vi "FlexMag - 24-03-2023.vi"() -> ()   [LabVIEW 2018] (continued)
                    n11930 = local read "ABORT"() -> (w17188:bool)
                    n11931 = case shown="False" w17188 {
                      frame False {
                        n11932 = while {
                          i -> [w17193]
                          stop <- w17194 stop-if-true
                          n11933 = Greater Or Equal?(x=w17193, y=100) -> (x >= y?=w17191:bool)
                          n11934 = case shown="True" w17191 {
                            frame False {
                            }
                            frame True {
                              n11935 = local write "Warning Message"("Transfer process canceled!\nCH3 Trns Bp Right coulnt't be closed" ("Warning Message")) -> ()
                              n11936 = local write "trns error"(TRUE ("TRNS error")) -> ()
                            }
                          }
                          n11937 = local read "CH3_Trns_BP_Right_DI"() -> (w17189:bool)
                          n11938 = case shown="True" w17189 {
                            tunnel: [TRUE ("CH1_Trns_BP_Left_DO") FALSE ("CH1_Trns_BP_Left_DO")] -> w17190
                            frame False {
                            }
                            frame True {
                              n11939 = local write "CH3_Trns_BP_Right_DO"(FALSE ("TRNS error")) -> ()
                              n11940 = Wait Until Next ms Multiple(millisecond multiple=u32 200) -> ()  [unwired: 1 out]
                            }
                          }
                          n11941 = local read "ch3-2 transfer"() -> (w17197:bool)
                          n11942 = local read "ABORT"() -> (w17196:bool)
                          n11943 = Not(x=w17197) -> (.not. x?=w17195:bool)
                          n11944 = Compound Arithmetic op=OR(w17190, w17196, w17195) -> (w17194:bool)
                        }
                      }
                      frame True {
                      }
                    }
                  }
                }
              }
              frame #43 {
                n11945 = local read "ch3-2 transfer"() -> (w17204:bool)
                n11946 = case shown="True" w17204 {
                  frame False {
                  }
                  frame True {
                    n11947 = local read "ABORT"() -> (w17205:bool)
                    n11948 = case shown="False" w17205 {
                      frame False {
                        n11949 = local write "trns 3-2 led 20"(TRUE ("trns 1-2 led 1")) -> ()
                        n11950 = Wait (ms)(milliseconds to wait=u32 100) -> ()  [unwired: 1 out]
                      }
                      frame True {
                      }
                    }
                  }
                }
              }
              frame #44 {
                n11951 = local read "ch3-2 transfer"() -> (w17208:bool)
                n11952 = case shown="True" w17208 {
                  frame False {
                  }
                  frame True {
                    n11953 = local read "ABORT"() -> (w17209:bool)
                    n11954 = case shown="False" w17209 {
                      frame False {
                        n11955 = stacked-sequence {
                          frame #0 {
                            n11956 = local read "ch3-2 transfer"() -> (w17210:bool)
                            n11957 = case shown="True" w17210 {
                              frame False {
                              }
                              frame True {
                                n11958 = local write "CH2_Trns_GV_Open_DO"(FALSE ("trns clear")) -> ()
                              }
                            }
                          }
                          frame #1 {
                            n11959 = while {
                              i -> [w17216]
                              stop <- w17217 stop-if-true
                              n11960 = Greater Or Equal?(x=w17216, y=600) -> (x >= y?=w17214:bool)
                              n11961 = case shown="True" w17214 {
                                frame False {
                                }
                                frame True {
                                n11962 = local write "Warning Message"("Transfer process canceled!\nCH2-CH3 Trns GV couldn't be closed" ("Warning Message")) -> ()
                                n11963 = local write "trns error"(TRUE ("TRNS error")) -> ()
                                }
                              }
                              n11964 = local read "CH2_Trns_Gv_Close_DI"() -> (w17212:bool)
                              n11965 = case shown="False" w17212 {
                                tunnel: [FALSE ("CH1_Trns_BP_Left_DO") TRUE ("CH1_Trns_BP_Left_DO")] -> w17213
                                frame False {
                                n11966 = local write "CH2_Trns_GV_Close_DO"(TRUE ("TRNS error")) -> ()
                                n11967 = Wait Until Next ms Multiple(millisecond multiple=u32 200) -> ()  [unwired: 1 out]
                                }
                                frame True {
                                }
                              }
                              n11968 = local read "ch3-2 transfer"() -> (w17220:bool)
                              n11969 = local read "ABORT"() -> (w17219:bool)
                              n11970 = Not(x=w17220) -> (.not. x?=w17218:bool)
                              n11971 = Compound Arithmetic op=OR(w17213, w17219, w17218) -> (w17217:bool)
                            }
                          }
                        }
                      }
                      frame True {
                      }
                    }
                  }
                }
              }
              frame #45 {
                n11972 = local read "ch3-2 transfer"() -> (w17227:bool)
                n11973 = case shown="True" w17227 {
                  frame False {
                  }
                  frame True {
                    n11974 = local read "ABORT"() -> (w17228:bool)
                    n11975 = case shown="False" w17228 {
                      frame False {
                        n11976 = local write "trns 3-2 led 21"(TRUE ("trns 1-2 led 1")) -> ()
                        n11977 = Wait (ms)(milliseconds to wait=u32 100) -> ()  [unwired: 1 out]
                      }
                      frame True {
                      }
                    }
                  }
                }
              }
              frame #46 {
                n11978 = local read "ch3-2 transfer"() -> (w17231:bool)
                n11979 = case shown="True" w17231 {
                  frame False {
                  }
                  frame True {
                    n11980 = local read "ABORT"() -> (w17232:bool)
                    n11981 = case shown="False" w17232 {
                      frame False {
                        n11982 = local read "target chamber"() -> (w17233:dbl)
                        n11983 = Equal?(x=w17233, y=2.0) -> (x = y?=w17234:bool)
                        n11984 = case shown="True" w17234 {
                          frame False {
                          }
                          frame True {
                            n11985 = stacked-sequence {
                              frame #0 {
                                n11986 = local read "ch3-2 transfer"() -> (w17236:bool)
                                n11987 = case shown="True" w17236 {
                                frame False {
                                }
                                frame True {
                                n11988 = local write "CH2_PetCool_Up_DO"(FALSE ("trns clear")) -> ()
                                }
                                }
                              }
                              frame #1 {
                                n11989 = while {
                                i -> [w17242]
                                stop <- w17243 stop-if-true
                                n11990 = Greater Or Equal?(x=w17242, y=300) -> (x >= y?=w17240:bool)
                                n11991 = case shown="True" w17240 {
                                frame False {
                                }
                                frame True {
                                n11992 = local write "Warning Message"("Transfer process canceled!\nCH2 Petcool couldn't be down" ("Warning Message")) -> ()
                                n11993 = local write "trns error"(TRUE ("TRNS error")) -> ()
                                }
                                }
                                n11994 = local read "CH2_PetCool_Down_DI"() -> (w17238:bool)
                                n11995 = case shown="False" w17238 {
                                tunnel: [FALSE ("CH1_Trns_BP_Left_DO") TRUE ("CH1_Trns_BP_Left_DO")] -> w17239
                                frame False {
                                n11996 = local write "CH2_PetCool_Down_DO"(TRUE ("TRNS error")) -> ()
                                n11997 = Wait Until Next ms Multiple(millisecond multiple=u32 200) -> ()  [unwired: 1 out]
                                }
                                frame True {
                                }
                                }
                                n11998 = local read "ch3-2 transfer"() -> (w17246:bool)
                                n11999 = local read "ABORT"() -> (w17245:bool)
                                n12000 = Not(x=w17246) -> (.not. x?=w17244:bool)
                                n12001 = Compound Arithmetic op=OR(w17239, w17245, w17244) -> (w17243:bool)
                                }
                              }
                            }
                          }
                        }
                      }
                      frame True {
                      }
                    }
                  }
                }
              }
              frame #47 {
                n12002 = local read "ch3-2 transfer"() -> (w17253:bool)
                n12003 = case shown="True" w17253 {
                  frame False {
                  }
                  frame True {
                    n12004 = local read "ABORT"() -> (w17254:bool)
                    n12005 = case shown="False" w17254 {
                      frame False {
                        n12006 = local write "trns 3-2 led 22"(TRUE ("trns 1-2 led 1")) -> ()
                        n12007 = Wait (ms)(milliseconds to wait=u32 100) -> ()  [unwired: 1 out]
                      }
                      frame True {
                      }
                    }
                  }
                }
              }
              frame #48 {
                n12008 = local read "ch3-2 transfer"() -> (w17257:bool)
                n12009 = case shown="True" w17257 {
                  frame False {
                  }
                  frame True {
                    n12010 = local read "ABORT"() -> (w17258:bool)
                    n12011 = case shown="False" w17258 {
                      frame False {
                        n12012 = local read "target chamber"() -> (w17260:dbl)
                        n12013 = Equal?(x=w17260, y=2.0) -> (x = y?=w17259:bool)
                        n12014 = case shown="True" w17259 {
                          frame False {
                          }
                          frame True {
                            n12015 = stacked-sequence {
                              frame #0 {
                                n12016 = local read "ch3-2 transfer"() -> (w17262:bool)
                                n12017 = case shown="True" w17262 {
                                frame False {
                                }
                                frame True {
                                n12018 = local write "CH2_SRV1_Piston_Back_DO"(FALSE ("trns clear")) -> ()
                                }
                                }
                              }
                              frame #1 {
                                n12019 = while {
                                i -> [w17268]
                                stop <- w17269 stop-if-true
                                n12020 = Greater Or Equal?(x=w17268, y=200) -> (x >= y?=w17266:bool)
                                n12021 = case shown="True" w17266 {
                                frame False {
                                }
                                frame True {
                                n12022 = local write "Warning Message"("Transfer process canceled!\nCH2 Servo Piston couldn't be forward" ("Warning Message")) -> ()
                                n12023 = local write "trns error"(TRUE ("TRNS error")) -> ()
                                }
                                }
                                n12024 = local read "CH2_SRV1_Piston_For_DI"() -> (w17264:bool)
                                n12025 = case shown="False" w17264 {
                                tunnel: [FALSE ("CH1_Trns_BP_Left_DO") TRUE ("CH1_Trns_BP_Left_DO")] -> w17265
                                frame False {
                                n12026 = local write "CH2_SRV1_Piston_For_DO"(TRUE ("TRNS error")) -> ()
                                n12027 = Wait Until Next ms Multiple(millisecond multiple=u32 200) -> ()  [unwired: 1 out]
                                }
                                frame True {
                                }
                                }
                                n12028 = local read "ch3-2 transfer"() -> (w17272:bool)
                                n12029 = local read "ABORT"() -> (w17271:bool)
                                n12030 = Not(x=w17272) -> (.not. x?=w17270:bool)
                                n12031 = Compound Arithmetic op=OR(w17265, w17271, w17270) -> (w17269:bool)
                                }
                              }
                            }
                          }
                        }
                      }
                      frame True {
                      }
                    }
                  }
                }
              }
              frame #49 {
                n12032 = local read "ch3-2 transfer"() -> (w17279:bool)
                n12033 = case shown="True" w17279 {
                  frame False {
                  }
                  frame True {
                    n12034 = local read "ABORT"() -> (w17280:bool)
                    n12035 = case shown="False" w17280 {
                      frame False {
                        n12036 = local write "trns 3-2 led 23"(TRUE ("trns 1-2 led 1")) -> ()
                        n12037 = Wait (ms)(milliseconds to wait=u32 100) -> ()  [unwired: 1 out]
                      }
                      frame True {
                      }
                    }
                  }
                }
              }
              frame #50 {
                n12038 = local read "ch3-2 transfer"() -> (w17283:bool)
                n12039 = case shown="True" w17283 {
                  frame False {
                  }
                  frame True {
                    n12040 = local read "ABORT"() -> (w17284:bool)
                    n12041 = case shown="False" w17284 {
                      frame False {
                        n12042 = disable-structure shown="Enabled" {
                          frame Disabled {
                            n12043 = stacked-sequence {
                              frame #0 {
                                n12044 = while {
                                i -> [w17289]
                                stop <- w17290 stop-if-true
                                n12045 = Greater Or Equal?(x=w17289, y=100) -> (x >= y?=w17287:bool)
                                n12046 = case shown="True" w17287 {
                                frame False {
                                }
                                frame True {
                                n12047 = local write "Warning Message"("Transfer process canceled!\nRight Slow Sensor problem" ("Warning Message")) -> ()
                                n12048 = local write "trns error"(TRUE ("TRNS error")) -> ()
                                }
                                }
                                n12049 = local read "Cnt_Right_Slow DI"() -> (w17285:bool)
                                n12050 = case shown="True" w17285 {
                                tunnel: [TRUE ("CH1_Trns_BP_Left_DO") FALSE ("CH1_Trns_BP_Left_DO")] -> w17286
                                frame False {
                                }
                                frame True {
                                n12051 = Wait Until Next ms Multiple(millisecond multiple=u32 200) -> ()  [unwired: 1 out]
                                n12052 = local write "Cnt_Right_Slow DO"(FALSE ("TRNS error")) -> ()
                                }
                                }
                                n12053 = local read "ch3-2 transfer"() -> (w17293:bool)
                                n12054 = local read "ABORT"() -> (w17292:bool)
                                n12055 = Not(x=w17293) -> (.not. x?=w17291:bool)
                                n12056 = Compound Arithmetic op=OR(w17286, w17292, w17291) -> (w17290:bool)
                                }
                              }
                              frame #1 {
                                n12057 = while {
                                i -> [w17304]
                                stop <- w17305 stop-if-true
                                n12058 = Greater Or Equal?(x=w17304, y=100) -> (x >= y?=w17302:bool)
                                n12059 = case shown="True" w17302 {
                                frame False {
                                }
                                frame True {
                                n12060 = local write "Warning Message"("Transfer process canceled!\nRight Limit Sensor problem" ("Warning Message")) -> ()
                                n12061 = local write "trns error"(TRUE ("TRNS error")) -> ()
                                }
                                }
                                n12062 = local read "Cnt_Right_Limit DI"() -> (w17300:bool)
                                n12063 = case shown="True" w17300 {
                                tunnel: [TRUE ("CH1_Trns_BP_Left_DO") FALSE ("CH1_Trns_BP_Left_DO")] -> w17301
                                frame False {
                                }
                                frame True {
                                n12064 = Wait Until Next ms Multiple(millisecond multiple=u32 200) -> ()  [unwired: 1 out]
                                n12065 = local write "Cnt_Right_Limit DO"(FALSE ("TRNS error")) -> ()
                                }
                                }
                                n12066 = local read "ch3-2 transfer"() -> (w17308:bool)
                                n12067 = local read "ABORT"() -> (w17307:bool)
                                n12068 = Not(x=w17308) -> (.not. x?=w17306:bool)
                                n12069 = Compound Arithmetic op=OR(w17301, w17307, w17306) -> (w17305:bool)
                                }
                              }
                              frame #2 {
                                n12070 = while {
                                i -> [w17319]
                                stop <- w17320 stop-if-true
                                n12071 = Greater Or Equal?(x=w17319, y=100) -> (x >= y?=w17317:bool)
                                n12072 = case shown="True" w17317 {
                                frame False {
                                }
                                frame True {
                                n12073 = local write "Warning Message"("Transfer process canceled!\nLeft Slow Sensor problem" ("Warning Message")) -> ()
                                n12074 = local write "trns error"(TRUE ("TRNS error")) -> ()
                                }
                                }
                                n12075 = local read "Cnt_Left_Slow DI"() -> (w17315:bool)
                                n12076 = case shown="True" w17315 {
                                tunnel: [TRUE ("CH1_Trns_BP_Left_DO") FALSE ("CH1_Trns_BP_Left_DO")] -> w17316
                                frame False {
                                }
                                frame True {
                                n12077 = Wait Until Next ms Multiple(millisecond multiple=u32 200) -> ()  [unwired: 1 out]
                                n12078 = local write "Cnt_Left_Slow DO"(FALSE ("TRNS error")) -> ()
                                }
                                }
                                n12079 = local read "ch3-2 transfer"() -> (w17323:bool)
                                n12080 = local read "ABORT"() -> (w17322:bool)
                                n12081 = Not(x=w17323) -> (.not. x?=w17321:bool)
                                n12082 = Compound Arithmetic op=OR(w17316, w17322, w17321) -> (w17320:bool)
                                }
                              }
                              frame #3 {
                                n12083 = while {
                                i -> [w17334]
                                stop <- w17335 stop-if-true
                                n12084 = Greater Or Equal?(x=w17334, y=100) -> (x >= y?=w17332:bool)
                                n12085 = case shown="True" w17332 {
                                frame False {
                                }
                                frame True {
                                n12086 = local write "Warning Message"("Transfer process canceled!\nLeft Limit Sensor problem" ("Warning Message")) -> ()
                                n12087 = local write "trns error"(TRUE ("TRNS error")) -> ()
                                }
                                }
                                n12088 = local read "Cnt_Left_Limit DI"() -> (w17330:bool)
                                n12089 = case shown="True" w17330 {
                                tunnel: [TRUE ("CH1_Trns_BP_Left_DO") FALSE ("CH1_Trns_BP_Left_DO")] -> w17331
                                frame False {
                                }
                                frame True {
                                n12090 = Wait Until Next ms Multiple(millisecond multiple=u32 200) -> ()  [unwired: 1 out]
                                n12091 = local write "Cnt_Left_Limit DO"(FALSE ("TRNS error")) -> ()
                                }
                                }
                                n12092 = local read "ch3-2 transfer"() -> (w17338:bool)
                                n12093 = local read "ABORT"() -> (w17337:bool)
                                n12094 = Not(x=w17338) -> (.not. x?=w17336:bool)
                                n12095 = Compound Arithmetic op=OR(w17331, w17337, w17336) -> (w17335:bool)
                                }
                              }
                            }
                          }
                          frame Enabled {
                            w17345 = FALSE ("CH4_SRV1_Piston_For_DO")
                            w17346 = FALSE ("CH4_SRV1_Piston_For_DO")
                            n12096 = local write "CH1_Right_Limit_DO"(w17346) -> ()
                            n12097 = local write "CH1_Right_Slow_DO"(w17346) -> ()
                            n12098 = local write "CH2_Right_Limit_DO"(w17346) -> ()
                            n12099 = local write "CH2_Right_Slow_DO"(w17346) -> ()
                            n12100 = local write "CH2_Left_Slow_DO"(w17346) -> ()
                            n12101 = local write "CH2_Left_Limit_DO"(w17346) -> ()
                            n12102 = Wait (ms)(milliseconds to wait=u32 2000) -> ()  [unwired: 1 out]
                            n12103 = local write "CH3_Right_Limit_DO"(w17345) -> ()
                            n12104 = local write "CH3_Right_Slow_DO"(w17345) -> ()
                            n12105 = local write "CH3_Left_Slow_DO"(w17345) -> ()
                            n12106 = local write "CH3_Left_Limit_DO"(w17345) -> ()
                            n12107 = local write "CH4_Left_Limit_DO"(w17345) -> ()
                            n12108 = local write "CH4_Left_Slow_DO"(w17345) -> ()
                          }
                        }
                      }
                      frame True {
                      }
                    }
                  }
                }
              }
              frame #51 {
                n12109 = local read "ch3-2 transfer"() -> (w17348:bool)
                n12110 = case shown="True" w17348 {
                  frame False {
                  }
                  frame True {
                    n12111 = local read "ABORT"() -> (w17349:bool)
                    n12112 = case shown="False" w17349 {
                      frame False {
                        n12113 = local write "trns 3-2 led 24"(TRUE ("trns 1-2 led 17")) -> ()
                        n12114 = Wait (ms)(milliseconds to wait=u32 100) -> ()  [unwired: 1 out]
                      }
                      frame True {
                      }
                    }
                  }
                }
              }
              frame #52 {
                n12115 = local read "ch3-2 transfer"() -> (w17352:bool)
                n12116 = case shown="True" w17352 {
                  frame False {
                  }
                  frame True {
                    n12117 = local read "ABORT"() -> (w17353:bool)
                    n12118 = case shown="False" w17353 {
                      frame False {
                        n12119 = local write "Buzzer DO"(TRUE ("trns 1-2 led 17")) -> ()
                        n12120 = Wait (ms)(milliseconds to wait=u32 3000) -> ()  [unwired: 1 out]
                        n12121 = local write "System Status"("CH3 to CH2  Transfer Completed" ("System Status")) -> ()
                      }
                      frame True {
                      }
                    }
                  }
                }
              }
              frame #53 {
                n12122 = local read "ch3-2 transfer"() -> (w17357:bool)
                n12123 = case shown="True" w17357 {
                  frame False {
                  }
                  frame True {
                    n12124 = local read "ABORT"() -> (w17358:bool)
                    n12125 = case shown="False" w17358 {
                      frame False {
                        w17359 = u16 2 items=["CH1"=1, "CH2"=2, "CH3"=3, "CH4"=4] ("cassette position selection")
                        w17360 = FALSE ("trns 1-2 led 17")
                        n12126 = Wait (ms)(milliseconds to wait=u32 1000) -> ()  [unwired: 1 out]
                        n12127 = local write "ch3-2 transfer"(FALSE ("trns 1-2 led 17")) -> ()
                        n12128 = local write "Buzzer DO"(FALSE ("trns 1-2 led 17")) -> ()
                        n12129 = local write "cassette position selection"(w17359) -> ()
                        n12130 = local write "System Status"("SEMI-AUTOMATIC MODE " ("System Status")) -> ()
                        n12131 = Not(x=w17360) -> (.not. x?=w17361:bool)
                        n12132 = local write "present location"(2.0 ("present location")) -> ()
                        n12133 = local write "casette_ch1_gui"(w17360) -> ()
                        n12134 = local write "casette_ch2_gui"(w17361) -> ()
                        n12135 = local write "casette_ch3_gui"(w17360) -> ()
                        n12136 = local write "casette_ch4_gui"(w17360) -> ()
                      }
                      frame True {
                      }
                    }
                  }
                }
              }
              frame #54 {
              }
            }
          }
          frame True {
          }
        }
      }
      frame 6 {
        n12137 = local read "ABORT"() -> (w17367:bool)
        n12138 = case shown="False" w17367 {
          frame False {
            n12139 = stacked-sequence {
              frame #0 {
                n12140 = local read "ch4-3 transfer"() -> (w17368:bool)
                n12141 = case shown="True" w17368 {
                  frame False {
                  }
                  frame True {
                    n12142 = local read "present location"() -> (w17371:dbl)
                    n12143 = Wait (ms)(milliseconds to wait=u32 100) -> ()  [unwired: 1 out]
                    n12144 = Equal?(x=w17371, y=4.0) -> (x = y?=w17372:bool)
                    n12145 = case shown="True" w17372 {
                      frame False {
                        n12146 = local write "trns error"(TRUE ("TRNS error")) -> ()
                        n12147 = local write "Warning Message"("Transfer process canceled!\nCassette is not in CH4" ("Warning Message")) -> ()
                      }
                      frame True {
                        n12148 = local write "System Status"("CH4 to CH3  Transfer in Progress" ("System Status")) -> ()
                      }
                    }
                  }
                }
              }
              frame #1 {
                n12149 = local read "ch4-3 transfer"() -> (w17376:bool)
                n12150 = case shown="True" w17376 {
                  frame False {
                  }
                  frame True {
                    n12151 = stacked-sequence {
                      frame #0 {
                        n12152 = local read "ABORT"() -> (w17377:bool)
                        n12153 = case shown="False" w17377 {
                          frame False {
                            n12154 = local write "trns pre check"(TRUE ("trns pre check")) -> ()
                          }
                          frame True {
                          }
                        }
                      }
                      frame #1 {
                        n12155 = Wait (ms)(milliseconds to wait=u32 1000) -> ()  [unwired: 1 out]
                      }
                      frame #2 {
                        n12156 = while {
                          i -> [w17385]
                          stop <- w17382 stop-if-true
                          # "10 min"
                          n12157 = local read "trns pre check"() -> (w17389:bool)
                          n12158 = local read "ch4-3 transfer"() -> (w17381:bool)
                          n12159 = local read "ABORT"() -> (w17383:bool)
                          n12160 = Greater Or Equal?(x=w17385, y=u32 2000 ("millisecond multiple")) -> (x >= y?=w17384:bool)
                          n12161 = Not(x=w17389) -> (.not. x?=w17388:bool)
                          n12162 = Not(x=w17381) -> (.not. x?=w17380:bool)
                          n12163 = Compound Arithmetic op=OR(w17384, w17388, w17383, w17380) -> (w17382:bool)
                          n12164 = Wait Until Next ms Multiple(millisecond multiple=u32 300) -> ()  [unwired: 1 out]
                        }
                      }
                    }
                  }
                }
              }
              frame #2 {
                n12165 = local read "ch4-3 transfer"() -> (w17390:bool)
                n12166 = case shown="True" w17390 {
                  frame False {
                  }
                  frame True {
                    n12167 = local read "trns V?"() -> (w17391:bool)
                    n12168 = case shown="False" w17391 {
                      frame False {
                        n12169 = stacked-sequence {
                          frame #0 {
                            n12170 = local read "ABORT"() -> (w17392:bool)
                            n12171 = case shown="False" w17392 {
                              frame False {
                                w17394 = FALSE ("CH1_CH_ATM_DO")
                                n12172 = local write "CH3_CH_ATM_DO"(w17394) -> ()
                                n12173 = local write "CH4_CH_ATM_DO"(w17394) -> ()
                                n12174 = Wait (ms)(milliseconds to wait=u32 3000) -> ()  [unwired: 1 out]
                              }
                              frame True {
                              }
                            }
                          }
                          frame #1 {
                            n12175 = while {
                              i -> [w17397]
                              stop <- w17398 stop-if-true
                              n12176 = Greater Or Equal?(x=w17397, y=200) -> (x >= y?=w17395:bool)
                              n12177 = case shown="True" w17395 {
                                frame False {
                                }
                                frame True {
                                n12178 = local write "Warning Message"("Transfer process canceled!\nChambers should be on Atmosphere Pressure" ("Warning Message")) -> ()
                                n12179 = local write "trns error"(TRUE ("TRNS error")) -> ()
                                }
                              }
                              n12180 = local read "CH3_CH_ATM_DI"() -> (w17402:bool)
                              n12181 = local read "CH4_CH_ATM_DI"() -> (w17401:bool)
                              n12182 = local read "ch4-3 transfer"() -> (w17404:bool)
                              n12183 = local read "ABORT"() -> (w17405:bool)
                              n12184 = Not(x=w17404) -> (.not. x?=w17403:bool)
                              n12185 = And(x=w17402, y=w17401) -> (x .and. y?=w17400:bool)
                              n12186 = Compound Arithmetic op=OR(w17400, w17405, w17403) -> (w17398:bool)
                              n12187 = Wait Until Next ms Multiple(millisecond multiple=u32 300) -> ()  [unwired: 1 out]
                            }
                          }
                        }
                      }
                      frame True {
                        n12188 = local read "ch3 ch pg torr"() -> (w17414:dbl)
                        n12189 = local read "ch4 ch pg torr"() -> (w17411:dbl)
                        n12190 = Greater Or Equal?(x=w17414, y=0.5) -> (x >= y?=w17410:bool)
                        n12191 = Greater Or Equal?(x=w17411, y=0.5) -> (x >= y?=w17409:bool)
                        n12192 = Or(x=w17410, y=w17409) -> (x .or. y?=w17408:bool)
                        n12193 = local write "trns error"(w17408) -> ()
                      }
                    }
                  }
                }
              }
              frame #3 {
                n12194 = local read "ch4-3 transfer"() -> (w17415:bool)
                n12195 = case shown="True" w17415 {
                  frame False {
                  }
                  frame True {
                    n12196 = local read "ABORT"() -> (w17416:bool)
                    n12197 = case shown="False" w17416 {
                      frame False {
                        n12198 = while {
                          i -> [w17421]
                          stop <- w17422 stop-if-true
                          n12199 = Greater Or Equal?(x=w17421, y=100) -> (x >= y?=w17419:bool)
                          n12200 = case shown="True" w17419 {
                            frame False {
                            }
                            frame True {
                              n12201 = local write "trns error"(TRUE ("TRNS error")) -> ()
                              n12202 = local write "Warning Message"("Transfer process canceled!\nCH3 Trns BP Left couln't be opened" ("Warning Message")) -> ()
                            }
                          }
                          n12203 = local read "CH3_Trns_BP_Left_DI"() -> (w17418:bool)
                          n12204 = case shown="False" w17418 {
                            tunnel: [FALSE ("CH1_Trns_BP_Left_DO") TRUE ("CH1_Trns_BP_Left_DO")] -> w17417
                            frame False {
                              n12205 = Wait Until Next ms Multiple(millisecond multiple=u32 200) -> ()  [unwired: 1 out]
                              n12206 = local write "CH3_Trns_BP_Left_DO"(TRUE ("CH1_Trns_BP_Left_DO")) -> ()
                            }
                            frame True {
                            }
                          }
                          n12207 = local read "ch4-3 transfer"() -> (w17425:bool)
                          n12208 = local read "ABORT"() -> (w17424:bool)
                          n12209 = Not(x=w17425) -> (.not. x?=w17423:bool)
                          n12210 = Compound Arithmetic op=OR(w17417, w17424, w17423) -> (w17422:bool)
                        }
                      }
                      frame True {
                      }
                    }
                  }
                }
              }
              frame #4 {
                n12211 = local read "ch4-3 transfer"() -> (w17432:bool)
                n12212 = case shown="True" w17432 {
                  frame False {
                  }
                  frame True {
                    n12213 = local read "ABORT"() -> (w17433:bool)
                    n12214 = case shown="False" w17433 {
                      frame False {
                        n12215 = local write "trns 4-3 led 1"(TRUE ("trns 1-2 led 1")) -> ()
                        n12216 = Wait (ms)(milliseconds to wait=u32 100) -> ()  [unwired: 1 out]
                      }
                      frame True {
                      }
                    }
                  }
                }
              }
              frame #5 {
                n12217 = local read "ch4-3 transfer"() -> (w17436:bool)
                n12218 = case shown="True" w17436 {
                  frame False {
                  }
                  frame True {
                    n12219 = local read "ABORT"() -> (w17437:bool)
                    n12220 = case shown="False" w17437 {
                      frame False {
                        n12221 = while {
                          i -> [w17442]
                          stop <- w17443 stop-if-true
                          n12222 = Greater Or Equal?(x=w17442, y=100) -> (x >= y?=w17440:bool)
                          n12223 = case shown="True" w17440 {
                            frame False {
                            }
                            frame True {
                              n12224 = local write "trns error"(TRUE ("TRNS error")) -> ()
                              n12225 = local write "Warning Message"("Transfer process canceled!\nCH2 Trns BP Right couln't be opened" ("Warning Message")) -> ()
                            }
                          }
                          n12226 = local read "CH4_Trns_BP_Right_DI"() -> (w17439:bool)
                          n12227 = case shown="False" w17439 {
                            tunnel: [FALSE ("CH1_Trns_BP_Left_DO") TRUE ("CH1_Trns_BP_Left_DO")] -> w17438
                            frame False {
                              n12228 = Wait Until Next ms Multiple(millisecond multiple=u32 200) -> ()  [unwired: 1 out]
                              n12229 = local write "CH4_Trns_BP_Right_DO"(TRUE ("CH1_Trns_BP_Left_DO")) -> ()
                            }
                            frame True {
                            }
                          }
                          n12230 = local read "ch4-3 transfer"() -> (w17446:bool)
                          n12231 = local read "ABORT"() -> (w17445:bool)
                          n12232 = Not(x=w17446) -> (.not. x?=w17444:bool)
                          n12233 = Compound Arithmetic op=OR(w17438, w17445, w17444) -> (w17443:bool)
                        }
                      }
                      frame True {
                      }
                    }
                  }
                }
              }
              frame #6 {
                n12234 = local read "ch4-3 transfer"() -> (w17453:bool)
                n12235 = case shown="True" w17453 {
                  frame False {
                  }
                  frame True {
                    n12236 = local read "ABORT"() -> (w17454:bool)
                    n12237 = case shown="False" w17454 {
                      frame False {
                        n12238 = local write "trns 4-3 led 2"(TRUE ("trns 1-2 led 1")) -> ()
                        n12239 = Wait (ms)(milliseconds to wait=u32 100) -> ()  [unwired: 1 out]
                      }
                      frame True {
                      }
                    }
                  }
                }
              }
              frame #7 {
                n12240 = local read "ch4-3 transfer"() -> (w17457:bool)
                n12241 = case shown="True" w17457 {
                  frame False {
                  }
                  frame True {
                    n12242 = local read "ABORT"() -> (w17458:bool)
                    n12243 = case shown="False" w17458 {
                      frame False {
                        n12244 = stacked-sequence {
                          frame #0 {
                            n12245 = local write "CH3_Trns_GV_Close_DO"(FALSE ("CH1_Trns_Gv_Close_DO")) -> ()
                            n12246 = Wait (ms)(milliseconds to wait=u32 100) -> ()  [unwired: 1 out]
                          }
                          frame #1 {
                            n12247 = while {
                              i -> [w17465]
                              stop <- w17466 stop-if-true
                              n12248 = Greater Or Equal?(x=w17465, y=600) -> (x >= y?=w17463:bool)
                              n12249 = case shown="True" w17463 {
                                frame False {
                                }
                                frame True {
                                n12250 = local write "trns error"(TRUE ("TRNS error")) -> ()
                                n12251 = local write "Warning Message"("Transfer process canceled!\nCH3-CH4 Trns GV couldn't be opened" ("Warning Message")) -> ()
                                }
                              }
                              n12252 = local read "CH3_Trns_Gv_Open_DI"() -> (w17462:bool)
                              n12253 = case shown="False" w17462 {
                                tunnel: [FALSE ("CH1_Trns_BP_Left_DO") TRUE ("CH1_Trns_BP_Left_DO")] -> w17461
                                frame False {
                                n12254 = local write "CH3_Trns_GV_Open_DO"(TRUE ("CH1_Trns_BP_Left_DO")) -> ()
                                n12255 = Wait Until Next ms Multiple(millisecond multiple=u32 200) -> ()  [unwired: 1 out]
                                }
                                frame True {
                                }
                              }
                              n12256 = local read "ch4-3 transfer"() -> (w17469:bool)
                              n12257 = local read "ABORT"() -> (w17468:bool)
                              n12258 = Not(x=w17469) -> (.not. x?=w17467:bool)
                              n12259 = Compound Arithmetic op=OR(w17461, w17468, w17467) -> (w17466:bool)
                            }
                          }
                        }
                      }
                      frame True {
                      }
                    }
                  }
                }
              }
              frame #8 {
                n12260 = local read "ch4-3 transfer"() -> (w17476:bool)
                n12261 = case shown="True" w17476 {
                  frame False {
                  }
                  frame True {
                    n12262 = local read "ABORT"() -> (w17477:bool)
                    n12263 = case shown="False" w17477 {
                      frame False {
                        n12264 = local write "trns 4-3 led 3"(TRUE ("trns 1-2 led 1")) -> ()
                        n12265 = Wait (ms)(milliseconds to wait=u32 100) -> ()  [unwired: 1 out]
                      }
                      frame True {
                      }
                    }
                  }
                }
              }
              frame #9 {
                n12266 = local read "ch4-3 transfer"() -> (w17480:bool)
                n12267 = case shown="True" w17480 {
                  frame False {
                  }
                  frame True {
                    n12268 = local read "ABORT"() -> (w17481:bool)
                    n12269 = case shown="False" w17481 {
                      frame False {
                        n12270 = while {
                          i -> [w17486]
                          stop <- w17487 stop-if-true
                          n12271 = Greater Or Equal?(x=w17486, y=100) -> (x >= y?=w17484:bool)
                          n12272 = case shown="True" w17484 {
                            frame False {
                            }
                            frame True {
                              n12273 = local write "trns error"(TRUE ("TRNS error")) -> ()
                              n12274 = local write "Warning Message"("Transfer process canceled!\nCH3 TGV Control Problem" ("Warning Message")) -> ()
                            }
                          }
                          n12275 = local read "CH3_TGV_Control_DI"() -> (w17483:bool)
                          n12276 = case shown="True" w17483 {
                            tunnel: [TRUE ("CH1_Trns_BP_Left_DO") FALSE ("CH1_Trns_BP_Left_DO")] -> w17482
                            frame False {
                            }
                            frame True {
                              n12277 = Wait Until Next ms Multiple(millisecond multiple=u32 200) -> ()  [unwired: 1 out]
                              n12278 = local write "CH3_TGV_Control_DO"(FALSE ("CH1_Trns_BP_Left_DO")) -> ()
                            }
                          }
                          n12279 = local read "ch4-3 transfer"() -> (w17490:bool)
                          n12280 = local read "ABORT"() -> (w17489:bool)
                          n12281 = Not(x=w17490) -> (.not. x?=w17488:bool)
                          n12282 = Compound Arithmetic op=OR(w17482, w17489, w17488) -> (w17487:bool)
                        }
                      }
                      frame True {
                      }
                    }
                  }
                }
              }
              frame #10 {
                n12283 = local read "ch4-3 transfer"() -> (w17497:bool)
                n12284 = case shown="True" w17497 {
                  frame False {
                  }
                  frame True {
                    n12285 = local read "ABORT"() -> (w17498:bool)
                    n12286 = case shown="False" w17498 {
                      frame False {
                        n12287 = local write "trns 4-3 led 4"(TRUE ("trns 1-2 led 1")) -> ()
                        n12288 = Wait (ms)(milliseconds to wait=u32 100) -> ()  [unwired: 1 out]
                      }
                      frame True {
                      }
                    }
                  }
                }
              }
              frame #11 {
                n12289 = local read "ch4-3 transfer"() -> (w17501:bool)
                n12290 = case shown="True" w17501 {
                  frame False {
                  }
                  frame True {
                    n12291 = local read "ABORT"() -> (w17502:bool)
                    n12292 = case shown="False" w17502 {
                      frame False {
                        n12293 = while {
                          i -> [w17507]
                          stop <- w17508 stop-if-true
                          n12294 = local read "CH1_Trns_Interlock_DI"() -> (w17503:bool)
                          n12295 = Greater Or Equal?(x=w17507, y=100) -> (x >= y?=w17505:bool)
                          n12296 = case shown="True" w17505 {
                            frame False {
                            }
                            frame True {
                              n12297 = local write "Warning Message"("Transfer process canceled!\nCH1 Interlock problem" ("Warning Message")) -> ()
                              n12298 = local write "trns error"(TRUE ("TRNS error")) -> ()
                            }
                          }
                          n12299 = case shown="False" w17503 {
                            tunnel: [w17512 TRUE ("CH1_Trns_BP_Left_DO")] -> w17504
                            frame False {
                              n12300 = local read "CH1_TGV_Control_DI"() -> (w17513:bool)
                              n12301 = case shown="False" w17513 {
                                tunnel: [FALSE ("CH1_Trns_BP_Left_DO") TRUE ("CH1_Trns_BP_Left_DO")] -> w17512
                                frame False {
                                n12302 = Wait Until Next ms Multiple(millisecond multiple=u32 200) -> ()  [unwired: 1 out]
                                n12303 = local write "CH1_TGV_Control_DO"(TRUE ("CH1_Trns_BP_Left_DO")) -> ()
                                }
                                frame True {
                                }
                              }
                            }
                            frame True {
                            }
                          }
                          n12304 = local read "ch4-3 transfer"() -> (w17511:bool)
                          n12305 = local read "ABORT"() -> (w17510:bool)
                          n12306 = Not(x=w17511) -> (.not. x?=w17509:bool)
                          n12307 = Compound Arithmetic op=OR(w17504, w17510, w17509) -> (w17508:bool)
                        }
                      }
                      frame True {
                      }
                    }
                  }
                }
              }
              frame #12 {
                n12308 = local read "ch4-3 transfer"() -> (w17521:bool)
                n12309 = case shown="True" w17521 {
                  frame False {
                  }
                  frame True {
                    n12310 = local read "ABORT"() -> (w17522:bool)
                    n12311 = case shown="False" w17522 {
                      frame False {
                        w17523 = TRUE ("CH4_Left_Limit_DO")
                        n12312 = local write "trns 4-3 led 5"(TRUE ("trns 1-2 led 1")) -> ()
                        n12313 = Wait (ms)(milliseconds to wait=u32 100) -> ()  [unwired: 1 out]
                        n12314 = local write "CH4_Left_Limit_DO"(w17523) -> ()
                        n12315 = local write "CH4_Left_Slow_DO"(w17523) -> ()
                      }
                      frame True {
                      }
                    }
                  }
                }
              }
              frame #13 {
                n12316 = local read "ch4-3 transfer"() -> (w17526:bool)
                n12317 = case shown="True" w17526 {
                  frame False {
                  }
                  frame True {
                    n12318 = local read "ABORT"() -> (w17527:bool)
                    n12319 = case shown="False" w17527 {
                      frame False {
                        n12320 = while {
                          i -> [w17532]
                          stop <- w17533 stop-if-true
                          n12321 = local read "CH3_Trns_Interlock_DI"() -> (w17528:bool)
                          n12322 = Greater Or Equal?(x=w17532, y=100) -> (x >= y?=w17530:bool)
                          n12323 = case shown="True" w17530 {
                            frame False {
                            }
                            frame True {
                              n12324 = local write "Warning Message"("Transfer process canceled!\nCH3 Interlock problem" ("Warning Message")) -> ()
                              n12325 = local write "trns error"(TRUE ("TRNS error")) -> ()
                            }
                          }
                          n12326 = case shown="False" w17528 {
                            tunnel: [w17537 TRUE ("CH1_Trns_BP_Left_DO")] -> w17529
                            frame False {
                              n12327 = local read "CH3_TGV_Control_DI"() -> (w17538:bool)
                              n12328 = case shown="False" w17538 {
                                tunnel: [FALSE ("CH1_Trns_BP_Left_DO") TRUE ("CH1_Trns_BP_Left_DO")] -> w17537
                                frame False {
                                n12329 = Wait Until Next ms Multiple(millisecond multiple=u32 200) -> ()  [unwired: 1 out]
                                n12330 = local write "CH3_TGV_Control_DO"(TRUE ("CH1_Trns_BP_Left_DO")) -> ()
                                }
                                frame True {
                                }
                              }
                            }
                            frame True {
                            }
                          }
                          n12331 = local read "ch4-3 transfer"() -> (w17536:bool)
                          n12332 = local read "ABORT"() -> (w17535:bool)
                          n12333 = Not(x=w17536) -> (.not. x?=w17534:bool)
                          n12334 = Compound Arithmetic op=OR(w17529, w17535, w17534) -> (w17533:bool)
                        }
                      }
                      frame True {
                      }
                    }
                  }
                }
              }
              frame #14 {
                n12335 = local read "ch4-3 transfer"() -> (w17546:bool)
                n12336 = case shown="True" w17546 {
                  frame False {
                  }
                  frame True {
                    n12337 = local read "ABORT"() -> (w17547:bool)
                    n12338 = case shown="False" w17547 {
                      frame False {
                        n12339 = local write "trns 4-3 led 6"(TRUE ("trns 1-2 led 1")) -> ()
                        n12340 = Wait (ms)(milliseconds to wait=u32 100) -> ()  [unwired: 1 out]
                      }
                      frame True {
                      }
                    }
                  }
                }
              }
              frame #15 {
                n12341 = local read "ch4-3 transfer"() -> (w17550:bool)
                n12342 = case shown="True" w17550 {
                  frame False {
                  }
                  frame True {
                    n12343 = local read "ABORT"() -> (w17551:bool)
                    n12344 = case shown="False" w17551 {
                      frame False {
                        n12345 = while {
                          i -> [w17556]
                          stop <- w17557 stop-if-true
                          n12346 = local read "CH4_Trns_Interlock_DI"() -> (w17552:bool)
                          n12347 = Greater Or Equal?(x=w17556, y=100) -> (x >= y?=w17554:bool)
                          n12348 = case shown="True" w17554 {
                            frame False {
                            }
                            frame True {
                              n12349 = local write "Warning Message"("Transfer process canceled!\nCH4 Interlock problem" ("Warning Message")) -> ()
                              n12350 = local write "trns error"(TRUE ("TRNS error")) -> ()
                            }
                          }
                          n12351 = case shown="False" w17552 {
                            tunnel: [w17561 TRUE ("CH1_Trns_BP_Left_DO")] -> w17553
                            frame False {
                              n12352 = local read "CH4_TGV_Control_DI"() -> (w17562:bool)
                              n12353 = case shown="False" w17562 {
                                tunnel: [FALSE ("CH1_Trns_BP_Left_DO") TRUE ("CH1_Trns_BP_Left_DO")] -> w17561
                                frame False {
                                n12354 = Wait Until Next ms Multiple(millisecond multiple=u32 200) -> ()  [unwired: 1 out]
                                n12355 = local write "CH4_TGV_Control_DO"(TRUE ("CH1_Trns_BP_Left_DO")) -> ()
                                }
                                frame True {
                                }
                              }
                            }
                            frame True {
                            }
                          }
                          n12356 = local read "ch4-3 transfer"() -> (w17560:bool)
                          n12357 = local read "ABORT"() -> (w17559:bool)
                          n12358 = Not(x=w17560) -> (.not. x?=w17558:bool)
                          n12359 = Compound Arithmetic op=OR(w17553, w17559, w17558) -> (w17557:bool)
                        }
                      }
                      frame True {
                      }
                    }
                  }
                }